vi "Main.vi"() -> ()   [LabVIEW 2020]
uses:
  System.Windows.Forms
  Global_Variable/Global.vi
  Database/Global1.vi
  Global_Variable/A131258.vi
  <userlib>/_MGI/Menu Building/MenuTypes/MenuStrip/MGI_MenuStrip.lvclass
  <userlib>/_MGI/Menu Building/MenuItemStatusChange/MGI_MenuItemStatusChange.lvclass
  Libraries/S7/S7.lvlib
panel:
  in  "产品更换":refnum<vi>
  in  "表格控件":string[][](table)
  out "上学状态":string
  in  "Andon":enum32{"未选择", "缺料报警", "质量报警", "故障报警"}(radio)
  out "PLC":bool
  in  "菜单":refnum<k24>(container)
  out "逆向空载":bool
  out "产品编号":string
  out "生产数量":i32
  out "合格数量":i32
  out "userStatus":string caption="用户状态"
  out "userName":string caption="用户名"
  out "connectionMode":string caption="联机类型"
  out "产品型号":string
  out "右工位曲线":bool
  out "左工位曲线":bool=TRUE
  out "振动NVH":bool
  out "备用试验1":bool
  out "备用试验2":bool
  out "手柄保持力":bool=TRUE caption="管柱保持力"
  out "锁紧/开启":bool
  out "手柄推拉力":bool caption="角度调节力"
  out "提示信息":string
  out "错误":bool
  out "时间字符串":string
  out "日期字符串":string
  out "自动":bool
  # "上下柱管压装"
  # "试验项目"
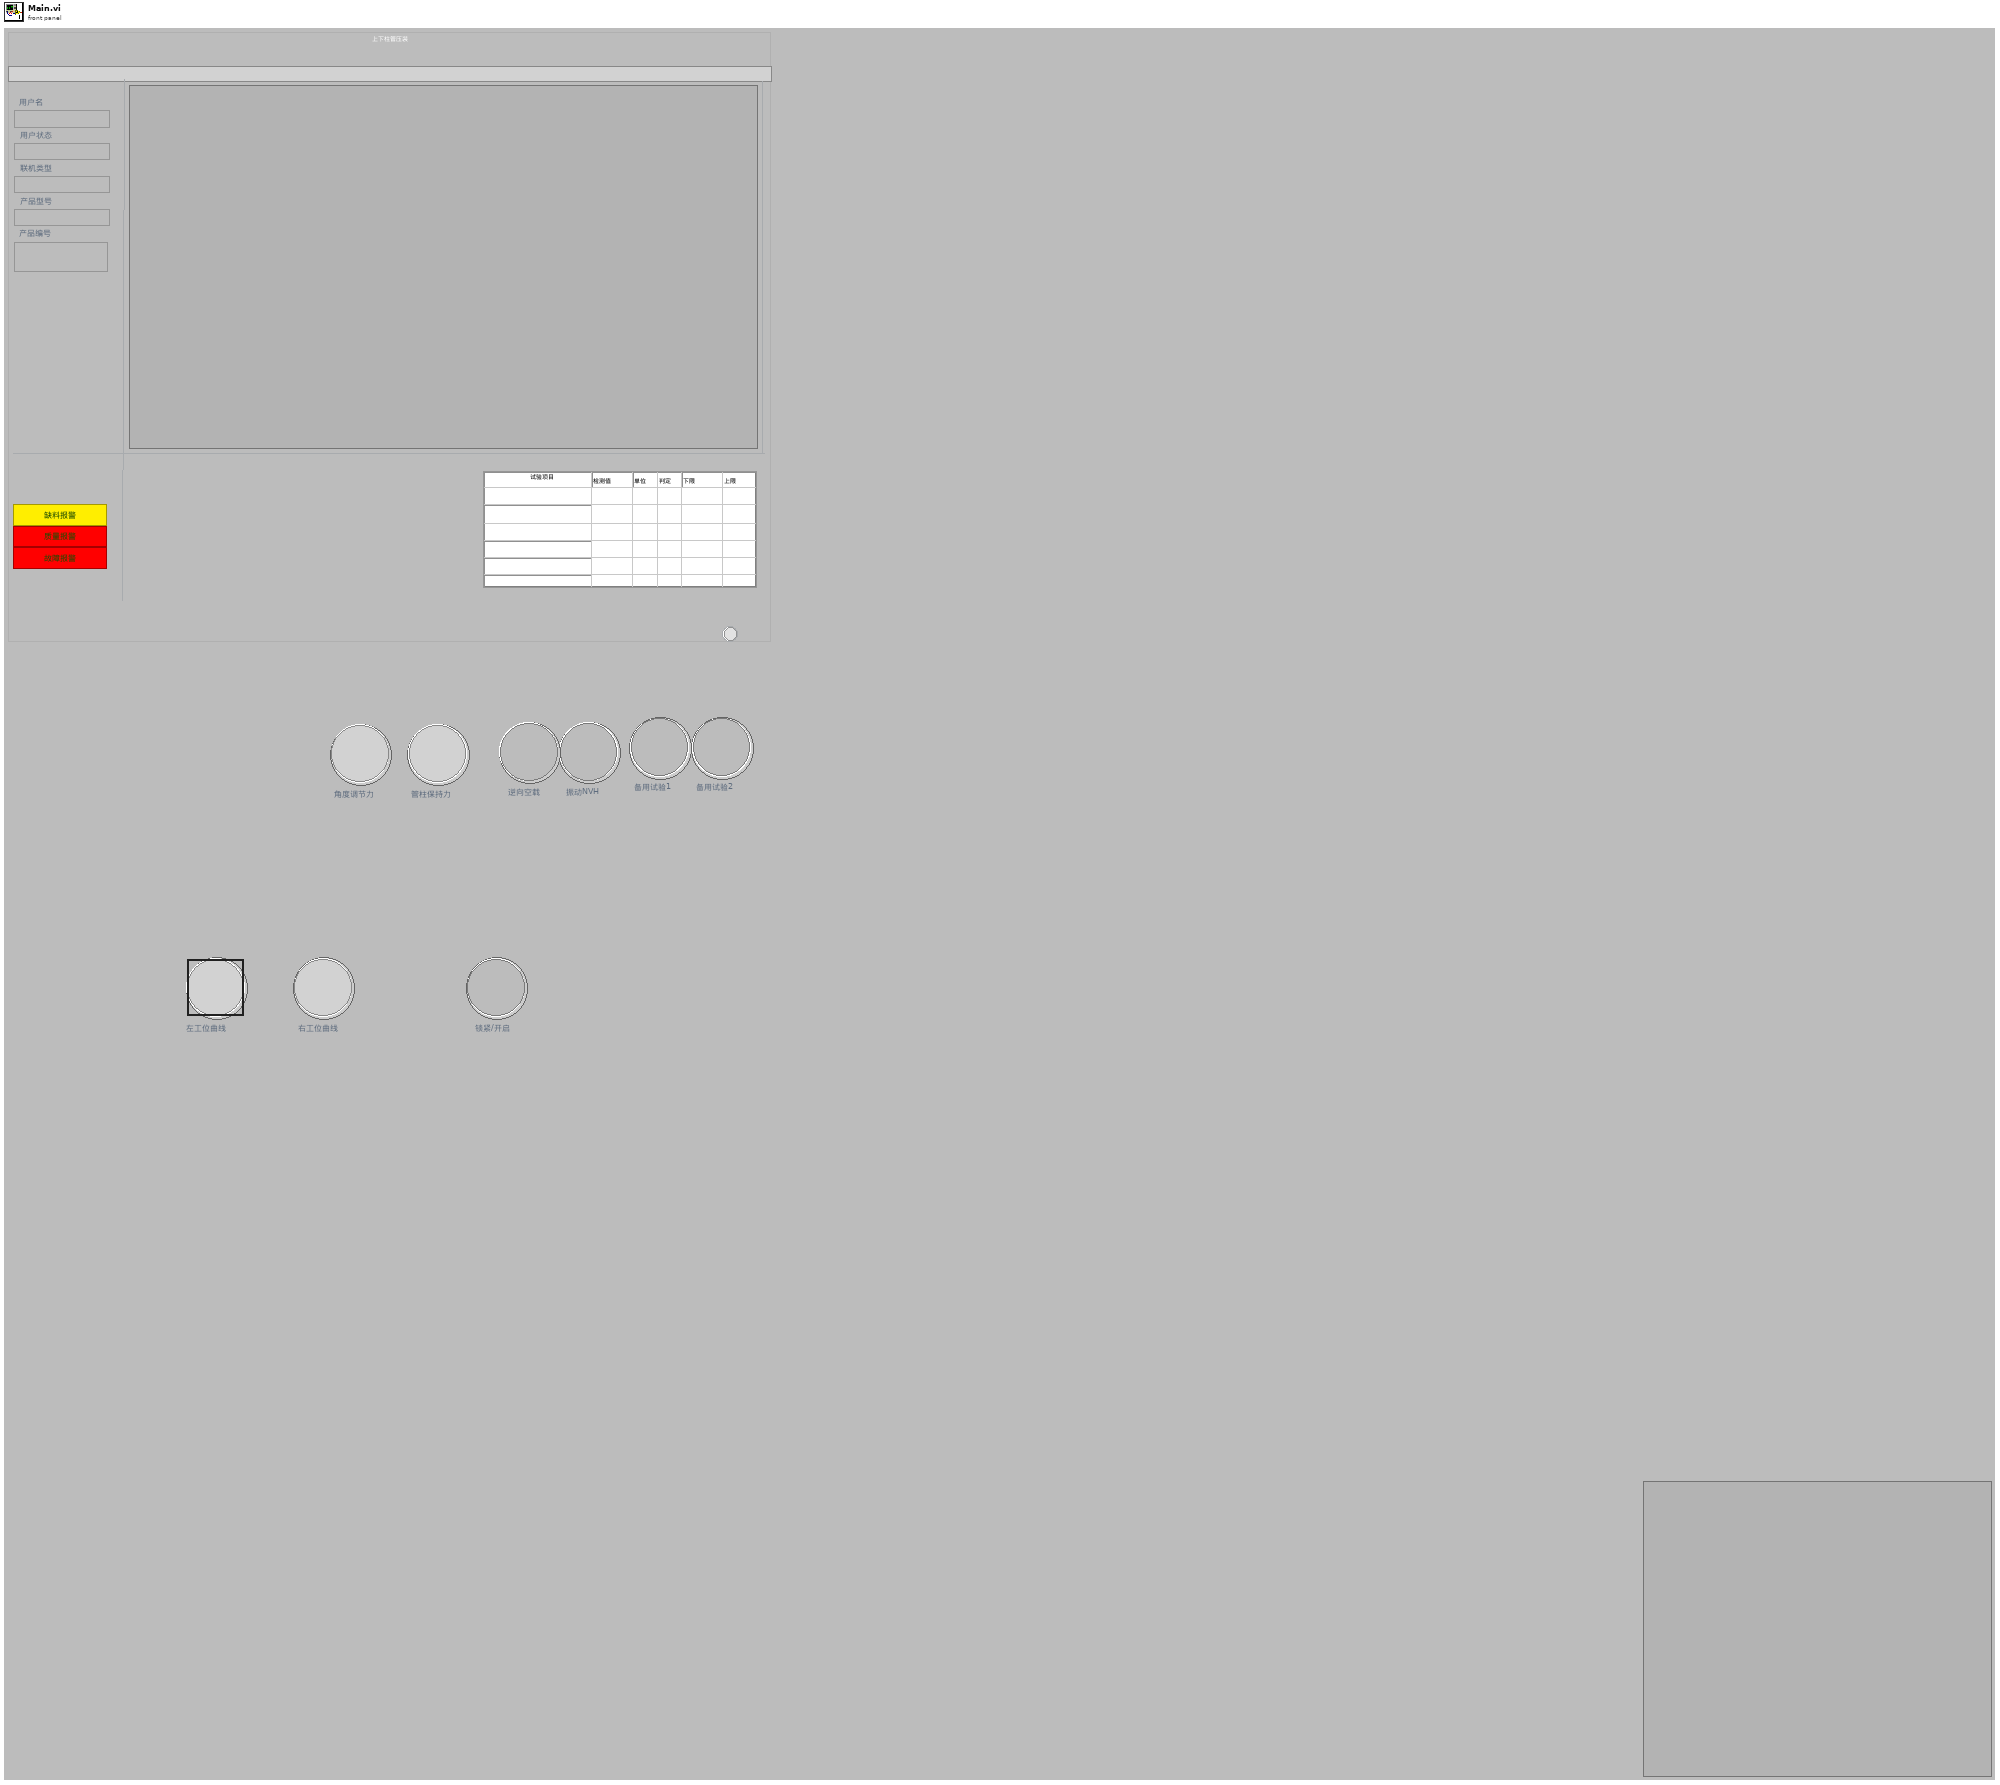
[diagram p1: front panel]
types:
  T1 = typedef "S7.lvlib/Broadcast Events--cluster.ctl" = cluster{"Module Did Init":refnum<user-event>, "Status Updated":refnum<user-event>, "Error Reported":refnum<user-event>, "Module Did Stop":refnum<user-event>, "Update Module Execution Status":refnum<user-event>}
  T2 = enum32{"左工位曲线", "右工位曲线", "手柄推拉力", "手柄保持力", "锁紧/开启", "逆向空载", "振动NVH"}
  T3 = enum32{"手柄锁紧力", "手柄开启力", "手柄推拉力", "手柄保持力", "锁紧/松开", "逆向空载", "振动NVH"}
  T4 = enum32{"手柄锁紧力", "手柄开启力", "手柄推拉力", "手柄保持力", "锁紧/开启", "逆向空载", "振动NVH"}
  T5 = enum32{"空载", "功能", "力特性", "电流特性", "传感器特性", "逆向空载", "振动NVH"}
  T6 = enum32{"Invalid", "Standard", "Closed", "Hidden", "Minimized", "Maximized"}
  T7 = cluster{"设备名称":string, "操作人员":string, "设备状态":enum16{"设备离线", "设备正常", "设备缺料", "设备故障", "质量报警"}, "附加信息":string}
  T8 = enum32{"invalid app kind", "Development System", "Run Time System", "Student Edition", "Embedded LabVIEW", "Evaluation", "Custom"}
  T9 = cluster{"用户编号":string, "用户名":string, "用户密码(密文)":string, "用户权限":string}
  T10 = cluster{"Core":cluster{"Current VI Reference":refnum<vi>, "Close Panel on Exit?":bool}, "Your Boolean data":bool, "Your string data":string}
  T11 = cluster{"Current VI Reference":refnum<vi>, "Close Panel on Exit?":bool}
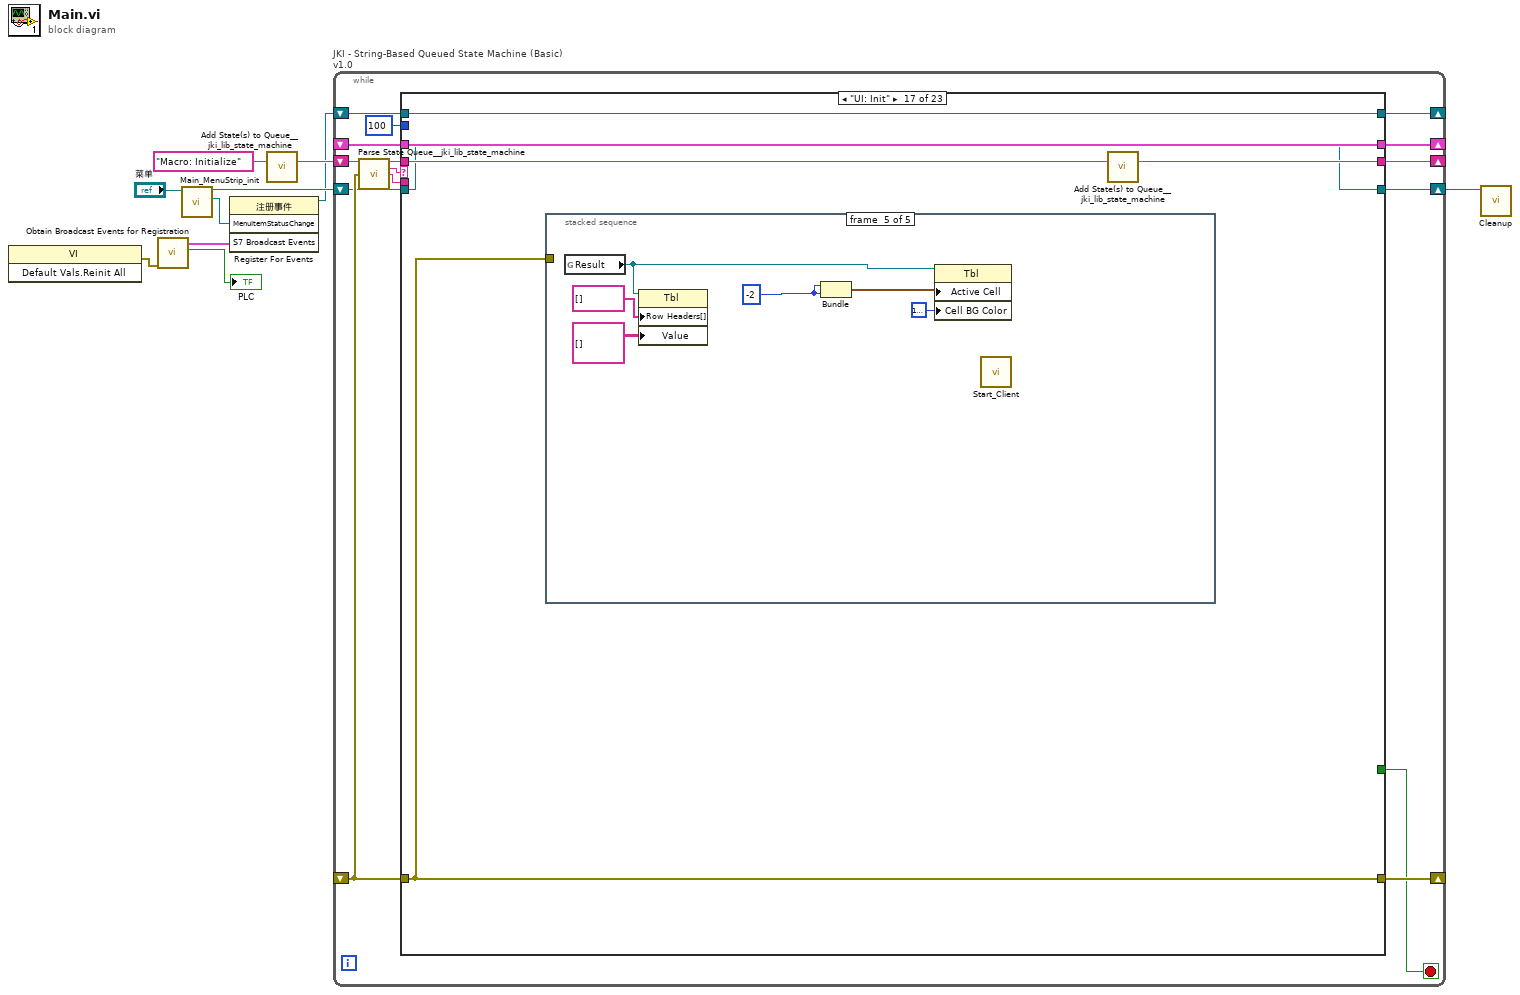
[diagram p0: block diagram]
diagram:
  n1 = invoke class="VI" method="Default Vals.Reinit All"() -> (error out=w3:errorcluster)  [unwired: 3 in, 2 out]
  n2 = call "Obtain Broadcast Events for Registration.vi"("error in (no error)"=w3) -> ("Already running?"=→"PLC":bool, "S7 Broadcast Events"=w1:T1)  [unwired: 8 in, 1 out]
  n3 = call "Main_MenuStrip_init.vi"("MenuStrip"="菜单") -> ("MenuItemStatusChange"=w5:refnum<user-event>, "Menu out"=w7:refnum<class "MGI_MenuStrip.lvclass">)  [unwired: 9 in]
  n4 = register-events(w5, w1) -> (reference out=w4:refnum<event-registration>)  [unwired: 2 in, 1 out]
  n5 = call <vilib>:"Add State(s) to Queue__jki_lib_state_machine.vi"("State(s) in (\"\")"="Macro: Initialize") -> ("States Out"=w10:string)  [unwired: 14 in]
  n6 = while "JKI - String-Based Queued State Machine (Basic) v1.0" {
    shift-right: [w19] -> _
    shift-left: _ -> [w18]
    shift-right: [w21] -> _
    shift-left: _ -> [w16]
    shift-right: [w20] -> _
    shift-left: w10 -> [w22]
    shift-right: [w14] -> w6
    shift-left: w7 -> [w15]
    shift-right: [w12] -> _
    shift-left: w4 -> [w11]
    stop <- w13 stop-if-true
    n7 = call <vilib>:"Parse State Queue__jki_lib_state_machine.vi"("State Queue"=w22, "Error In (no error)"=w16) -> ("Remaining States"=w24:string, "Current State"=w25:string, "Arguments"=w23:string)  [unwired: 11 in]
    n8 = case shown="\"UI: Init\"" w25 {
      selector: w25 -> [_ _ w269 _ _ _ _ _ _ _ _ _ _ _ _ _ _ _ _ _ _ _ _]
      tunnel: w24 -> [w36 w266 w273 w293 w301 w308 w314 w318 w324 w330 w336 w345 w356 w364 w370 w377 w401 w438 w446 w459 w487 w494 w506]
      tunnel: w23 -> [_ _ _ _ _ _ _ _ _ _ _ _ _ _ _ _ _ _ w441 w453 _ _ _]
      tunnel: w18 -> [w34 w263 w271 w284 w298 w306 w311 w319 w327 w333 w339 w342 _ w359 w367 w375 w399 w435 w444 w455 w484 w491 w503]
      tunnel: [w33 w264 w275 w290 errorcluster {"status"=FALSE, "code"=0, "source"=""} ("error out") w305 w312 w316 w321 w329 w335 w343 w353 w360 w368 w374 w397 w436 w442 w456 w485 w492 w504] -> w21
      tunnel: w16 -> [w32 w264 w274 w290 w297 w305 w312 w316 w322 w329 w335 w343 w353 w361 w368 w371 w397 w436 w443 w457 w485 w492 w504]
      tunnel: [w35 w265 w272 w292 w300 w307 w313 w318 w325 w331 w337 w344 w355 w363 w369 w376 w400 w437 w445 w458 w486 w493 w505] -> w20
      tunnel: [w31 w263 w271 w291 w298 w306 w311 w319 w327 w333 w339 w342 w354 w359 w367 w375 w399 w435 w444 w455 w484 w491 w503] -> w19
      tunnel: 100 ("Timeout") -> [w30 _ _ _ _ _ _ _ _ _ _ _ _ _ _ _ _ _ _ _ _ _ _]
      tunnel: w15 -> [w29 w262 w268 w281 w295 w304 w310 w317 w326 w332 w338 w341 w348 w358 w366 w373 w398 w434 w440 w452 w483 w489 w496]
      tunnel: [w28 w262 w268 w281 w295 w304 w310 w317 w326 w332 w338 w341 w348 w358 w366 w373 w398 w434 w440 w452 w483 w489 w496] -> w14
      tunnel: [_ _ _ _ _ TRUE _ _ _ _ _ _ _ _ _ _ _ _ _ _ _ _ _] -> w13
      tunnel: [w26 w261 w267 w280 w294 w302 w309 w320 w323 w328 w334 w340 w349 w357 w365 w372 w396 w431 w439 w451 w482 w488 w495] -> w12
      tunnel: w11 -> [w27 w261 w267 w280 w294 w302 w309 w320 w323 w328 w334 w340 w349 w357 w365 w372 w396 w431 w439 w451 w482 w488 w495]
      frame "", "Event Structure", "Idle" {
        n9 = event shown="[8] <S7 Broadcast Events.Error Reported>: 用户事件" {
          selector: w27 -> [w39 w58 w70 w141 w162 w170 w178 w185 w192 w193 w200 w211 _]
          dyn-events: [w39 w58 w70 w141 w152 w170 w178 w185 w192 w193 w200 w211 _] -> w26
          timeout: w30 -> [_ _ _ _ _ _ _ _ _ _ _ _ _]
          tunnel: w36 -> [w49 w61 w79 w138 w151 w167 w175 w182 w189 w197 w207 w210 w255]
          tunnel: [w48 w60 w77 w139 w151 w169 w177 w184 w191 w198 w206 w209 w255] -> w35
          tunnel: w34 -> [w47 w62 w78 w140 w153 w168 w176 w183 w190 w199 w204 w214 w256]
          tunnel: [w40 w59 w80 w136 w154 w165 w173 w180 w187 w196 w205 w213 w253] -> w33
          tunnel: w32 -> [w40 w59 w80 w136 w155 w165 w173 w180 _ w196 w205 w213 w253]
          tunnel: [w47 w62 w78 w140 w153 w168 w176 w183 w190 w199 w204 w214 w256] -> w31
          tunnel: w29 -> [w38 _ w73 w137 w150 w166 w174 w181 w188 _ _ _ w254]
          tunnel: [w38 _ w73 w137 w150 w166 w174 w181 w188 _ _ _ w254] -> w28
          event Timeout {
            (unwired) "" ("CODE_ID")
            n10 = event-data() -> ()  [unwired: 1 in, 1 out]
            n11 = Format Date/Time String(time format string (%c)="%H:%M ") -> (date/time string=→"时间字符串":string)  [unwired: 2 in]
            n12 = Format Date/Time String(time format string (%c)="%Y年%m月%d日") -> (date/time string=→"日期字符串":string)  [unwired: 2 in]
            n13 = global read "Global.vi" "追溯码"() -> (→"产品编号":string)
            n14 = call <vilib>:"Add State(s) to Queue__jki_lib_state_machine.vi"("State(s) in (\"\")"=w49) -> ("States Out"=w48:string)  [unwired: 14 in]
            n15 = global read "Global.vi" "合格数量"() -> (→"合格数量":i32)
            n16 = global read "Global.vi" "生产数量"() -> (→"生产数量":i32)
          }
          event "左工位曲线", "右工位曲线", "手柄推拉力", "手柄保持力", "锁紧/开启", "振动NVH", "逆向空载": Mouse Down {
            w50 = refnum<user-event> refnum items=["左工位曲线", "右工位曲线", "手柄推拉力", "手柄保持力", "锁紧/开启", "逆向空载", "振动NVH"] ("试验项_Event")
            n17 = event-data() -> ("CtlRef"=w54:refnum<vi>)  [unwired: 1 in]
            n18 = property class="Bool (严格)"(reference=w54) -> ("Label.Text"=w53:string)  [unwired: 1 in, 2 out]
            n19 = vi-ref "Auto.vi"() -> (w56:refnum<vi>)
            n20 = case shown="\"右工位曲线\"" w53 {
              tunnel: [T2."左工位曲线" ("试验项") T2."右工位曲线" ("试验项") T3."手柄推拉力" ("事件数据") T3."手柄保持力" ("事件数据") T4."锁紧/开启" ("事件数据") T5."逆向空载" ("事件数据") T5."振动NVH" ("事件数据")] -> w51
              frame "左工位曲线", Default {
              }
              frame "右工位曲线" {
              }
              frame "手柄推拉力" {
              }
              frame "手柄保持力" {
              }
              frame "锁紧/开启" {
              }
              frame "逆向空载" {
              }
              frame "振动NVH" {
              }
            }
            n21 = invoke class="VI" method="Ctrl Val.Get"(reference=w56, "Control Name"="试验项_Event" ("控件名")) -> ("Get Control Value Variant"=w55:variant)  [unwired: 2 in, 3 out]
            n22 = Variant To Data(type=w50, Variant=w55) -> (data=w52:refnum<user-event>)  [unwired: 1 in, 1 out]
            n23 = Generate User Event(user event=w52, event data cluster=w51) -> ()  [unwired: 2 in, 2 out]
            n24 = call <vilib>:"Add State(s) to Queue__jki_lib_state_machine.vi"("State(s) in (\"\")"=w61) -> ("States Out"=w60:string)  [unwired: 14 in]
          }
          event User Event {
            n25 = event-data() -> ("StatusChange"=w71:refnum<class "MGI_MenuItemStatusChange.lvclass">)  [unwired: 1 in]
            n26 = call <userlib>:"BasicInfo.vi"("MGI_MenuItemStatusChange in"=w71) -> ("Enabled?"=w74:bool, "Checked?"=w75:bool, "Tag"=w76:string)  [unwired: 7 in, 1 out]
            n27 = case shown="\"退出\"" w76 {
              tunnel: w75 -> [_ _ _ _ _ _ _ _ _ _ _ _ _ _ _]
              tunnel: w74 -> [_ _ _ _ _ _ _ _ _ _ _ _ _ _ _]
              tunnel: [_ _ "S7: Stop\nCAN: Stop\nMacro: Exit" _ _ _ _ _ _ _ _ _ _ _ _] -> w72
              frame "假", Default {
              }
              frame "数据库配置" {
                n28 = global read "Global1.vi" "用户信息"() -> (w81:T9)
                n29 = Unbundle By Name(w81) -> ("用户权限"=w82:string)
                n30 = case shown="\"系统管理员\"" w82 {
                  frame Default {
                    n31 = One Button Dialog(message="权限不足！" ("消息")) -> ()  [unwired: 1 in, 1 out]
                  }
                  frame "系统管理员" {
                    n32 = vi-ref "数据库配置.vi"() -> (w85:refnum<vi>)
                    n33 = call "CallVI.vi"("VI引用"=w85, "状态"=T6."Standard") -> ()  [unwired: 11 in, 3 out]
                  }
                }
              }
              frame "退出" {
                n34 = global write "Global.vi" "程序关闭"(TRUE ("程序关闭")) -> ()
                n35 = call "Close_Client.vi"() -> ()  [unwired: 12 in]
              }
              frame "手动控制" {
                n36 = global read "Global1.vi" "用户信息"() -> (w88:T9)
                n37 = Unbundle By Name(w88) -> ("用户权限"=w89:string)
                n38 = case shown="\"班组长\", \"系统管理员\"" w89 {
                  frame Default {
                    n39 = One Button Dialog(message="权限不足！" ("消息")) -> ()  [unwired: 1 in, 1 out]
                  }
                  frame "班组长", "系统管理员" {
                    n40 = vi-ref "111_IO.vi"() -> (w92:refnum<vi>)
                    n41 = call "CallVI.vi"("VI引用"=w92, "状态"=T6."Standard") -> ()  [unwired: 11 in, 3 out]
                  }
                }
              }
              frame "半自动控制" {
                n42 = disable-structure shown="启用" {
                  frame Disabled {
                    n43 = shared-variable "我的电脑\\Global.lvlib\\操作者权限"() -> (w93:string)  [unwired: 1 in, 1 out]
                    n44 = case shown="\"班组长\", \"系统管理员\"" w93 {
                      frame Default {
                        n45 = One Button Dialog(message="权限不足！" ("消息")) -> ()  [unwired: 1 in, 1 out]
                      }
                      frame "班组长", "系统管理员" {
                        n46 = call "CallVI.vi"("VI引用"=refnum<vi> refnum, "状态"=T6."Maximized") -> ()  [unwired: 11 in, 3 out]
                      }
                    }
                  }
                  frame Enabled {
                    n47 = One Button Dialog(message="当前设备不具备半自动功能！" ("消息")) -> ()  [unwired: 1 in, 1 out]
                  }
                }
              }
              frame "产品管理" {
                n48 = vi-ref "Config.vi"() -> (w99:refnum<vi>)
                n49 = call "CallVI.vi"("VI引用"=w99, "状态"=T6."Standard") -> ()  [unwired: 11 in, 3 out]
              }
              frame "系统配置" {
                n50 = global read "Global1.vi" "用户信息"() -> (w100:T9)
                n51 = Unbundle By Name(w100) -> ("用户权限"=w101:string)
                n52 = case shown="\"班组长\", \"系统管理员\"" w101 {
                  frame Default {
                    n53 = One Button Dialog(message="权限不足！" ("消息")) -> ()  [unwired: 1 in, 1 out]
                  }
                  frame "班组长", "系统管理员" {
                    n54 = vi-ref "111_Setting.vi"() -> (w104:refnum<vi>)
                    n55 = call "CallVI.vi"("VI引用"=w104, "状态"=T6."Standard") -> ()  [unwired: 11 in, 3 out]
                  }
                }
              }
              frame "用户管理" {
                n56 = global read "Global1.vi" "用户信息"() -> (w105:T9)
                n57 = Unbundle By Name(w105) -> ("用户权限"=w106:string)
                n58 = case shown="\"系统管理员\"" w106 {
                  frame Default {
                    n59 = One Button Dialog(message="权限不足！" ("消息")) -> ()  [unwired: 1 in, 1 out]
                  }
                  frame "系统管理员" {
                    n60 = vi-ref "User_manager.vi"() -> (w109:refnum<vi>)
                    n61 = call "CallVI.vi"("VI引用"=w109, "状态"=T6."Standard") -> ()  [unwired: 11 in, 3 out]
                  }
                }
              }
              frame "编码规则" {
                n62 = global read "Global1.vi" "用户信息"() -> (w110:T9)
                n63 = Unbundle By Name(w110) -> ("用户权限"=w111:string)
                n64 = case shown="\"班组长\", \"工艺管理员\", \"系统管理员\"" w111 {
                  frame Default {
                    n65 = One Button Dialog(message="权限不足！" ("消息")) -> ()  [unwired: 1 in, 1 out]
                  }
                  frame "班组长", "工艺管理员", "系统管理员" {
                    n66 = vi-ref "编码规则设置.vi"() -> (w114:refnum<vi>)
                    n67 = call "CallVI.vi"("VI引用"=w114, "状态"=T6."Standard") -> ()  [unwired: 11 in, 3 out]
                  }
                }
              }
              frame "易损件管理" {
                n68 = vi-ref "易损件管理.vi"() -> (w116:refnum<vi>)
                n69 = call "CallVI.vi"("VI引用"=w116, "状态"=T6."Standard") -> ()  [unwired: 11 in, 3 out]
              }
              frame "物料批次管理" {
                n70 = vi-ref "批次管理.vi"() -> (w118:refnum<vi>)
                n71 = call "CallVI.vi"("VI引用"=w118, "状态"=T6."Standard") -> ()  [unwired: 11 in, 3 out]
              }
              frame "报表" {
                n72 = call "文件对话框"("start path"=path "D:/report", "prompt"="打开报表", "pattern (all files)"="*.doc;*.docx", "pattern label"="Word 文档") -> ("selected path"=w119:path, "error out"=w120:errorcluster)  [unwired: 8 in, 2 out]
                n73 = case shown="无错误" w120 {
                  selector: w120 -> [w126 w128]
                  tunnel: w119 -> [w127 _]
                  frame No Error {
                    w125 = 1 items=["Normal", "Maximize", "Minimize"] ("cpubbs_WindowState")
                    n74 = call "Open_Word.vi"("File Path"=w127, "cpubbs_WindowState"=w125, "错误输入（无错误）"=w126) -> ()  [unwired: 12 in, 1 out]
                  }
                  frame Error {
                    n75 = call <vilib>:"Clear Errors.vi"("error in (no error)"=w128) -> ()  [unwired: 5 in, 2 out]
                  }
                }
              }
              frame "报警信息" {
                n76 = vi-ref "报警信息.vi"() -> (w130:refnum<vi>)
                n77 = call "CallVI.vi"("VI引用"=w130, "状态"=T6."Standard") -> ()  [unwired: 11 in, 3 out]
              }
              frame "关于" {
                n78 = vi-ref "About.vi"() -> (w132:refnum<vi>)
                n79 = call "CallVI.vi"("VI引用"=w132, "状态"=T6."Standard") -> ()  [unwired: 11 in, 3 out]
              }
              frame "操作演示" {
                n80 = call <vilib>:"Application Directory.vi"() -> ("Application Directory"=w135:path)
                n81 = Build Path(base path=w135, name or relative path="操作演示" ("名称或相对路径")) -> (appended path=w134:path)
                n82 = call "自动播放ppt.vi"("路径"=w134) -> ()  [unwired: 10 in, 1 out]
              }
            }
            n83 = call <vilib>:"Add State(s) to Queue__jki_lib_state_machine.vi"("State(s) in (\"\")"=w79, "State(s) at Back (\"\")"=w72) -> ("States Out"=w77:string)  [unwired: 13 in]
          }
          event "自动": Mouse Down {
            n84 = event-data() -> ()  [unwired: 1 in, 1 out]
            n85 = disable-structure shown="禁用" {
              frame Disabled {
                n86 = local read "自动"() -> (w142:bool)
                n87 = case shown="假" w142 {
                  frame False {
                    n88 = call "设备状态.vi"() -> ("Status_Read"=w143:i16)  [unwired: 11 in]
                    n89 = case shown="5" w143 {
                      frame 0, Default {
                        n90 = One Button Dialog(message="请复位！" ("消息")) -> ()  [unwired: 1 in, 1 out]
                      }
                      frame 5 {
                      }
                    }
                  }
                  frame True {
                    n91 = Two Button Dialog(message="确定要退出自动？" ("消息")) -> (T button?=w145:bool)  [unwired: 2 in]
                    n92 = case shown="真" w145 {
                      frame False {
                      }
                      frame True {
                        n93 = vi-ref "Auto.vi"() -> (w149:refnum<vi>)
                        n94 = invoke class="VI" method="Ctrl Val.Set"(reference=w149, "Control Name"="STEP" ("控件名"), "Value"="退出自动" ("控件名")) -> ()  [unwired: 2 in, 5 out]
                      }
                    }
                  }
                }
              }
              frame Enabled {
              }
            }
            n95 = call <vilib>:"Add State(s) to Queue__jki_lib_state_machine.vi"("State(s) in (\"\")"=w138) -> ("States Out"=w139:string)  [unwired: 14 in]
          }
          event "PLC": Value Change; "PLC": Mouse Down {
            n96 = event-data() -> ()  [unwired: 1 in, 4 out]
            n97 = call "Start Module.vi"("error in (no error)"=w155) -> ("error out"=w158:errorcluster, "Wait for Event Sync?"=w160:bool, "S7 Broadcast Events"=w161:T1, "Module Was Already Running?"=w163:bool)  [unwired: 7 in]
            n98 = local write "PLC"(w163) -> ()
            n99 = register-events(reference=w162, error in=w158, w161) -> (reference out=w152:refnum<event-registration>, error out=w164:errorcluster)  [unwired: 1 in]
            n100 = call "Synchronize Module Events.vi"("error in (no error)"=w164, "Wait for Event Sync?"=w160) -> ("error out"=w159:errorcluster)  [unwired: 9 in]
            n101 = call "Init S7 Link.vi"("error in (no error)"=w159, "超时"=500, "IP"="192.168.0.181") -> ("error out"=w154:errorcluster)  [unwired: 8 in]
          }
          event User Event {
            n102 = event-data() -> ("Init?"=w171:bool)  [unwired: 1 in, 5 out]
            n103 = local write "PLC"(w171) -> ()
            n104 = call <vilib>:"Add State(s) to Queue__jki_lib_state_machine.vi"("State(s) in (\"\")"=w167) -> ("States Out"=w169:string)  [unwired: 14 in]
          }
          event User Event {
            n105 = event-data() -> ()  [unwired: 1 in, 7 out]
            n106 = local write "PLC"(FALSE ("PLC")) -> ()
            n107 = call <vilib>:"Add State(s) to Queue__jki_lib_state_machine.vi"("State(s) in (\"\")"=w175) -> ("States Out"=w177:string)  [unwired: 14 in]
          }
          event User Event {
            n108 = event-data() -> ("Running?"=w179:bool)  [unwired: 1 in, 4 out]
            n109 = local write "PLC"(w179) -> ()
            n110 = call <vilib>:"Add State(s) to Queue__jki_lib_state_machine.vi"("State(s) in (\"\")"=w182) -> ("States Out"=w184:string)  [unwired: 14 in]
          }
          event User Event {
            n111 = event-data() -> ("Error"=w187:errorcluster)  [unwired: 1 in, 6 out]
            n112 = call <vilib>:"Add State(s) to Queue__jki_lib_state_machine.vi"("State(s) in Front (\"\")"="S7: Initialize\nIdle", "State(s) in (\"\")"=w189) -> ("States Out"=w191:string)  [unwired: 13 in]
          }
          event "错误": Mouse Down {
            n113 = event-data() -> ()  [unwired: 1 in, 8 out]
            n114 = vi-ref "报警信息.vi"() -> (w195:refnum<vi>)